vi "Main Test.vi"() -> ()   [LabVIEW 2020]
uses:
  Mete.ctl
  R.ctl
  P.ctl
  N.ctl
  D.ctl
  STOP.ctl
  Odo Velocity.ctl
  Gas.ctl
  Set-.ctl
  Set+.ctl
  Cru.ctl
  Dis.ctl
  CharRPM.ctl
  CharODO.ctl
  Brake.ctl
  Limit.ctl
  SET+LIMIT.ctl
  SET-LIMIT.ctl
panel:
  out "Image":T1(plugin-control)
  out "Boolean":T2
  in  "LIMIT-":T3
  in  "LIMT+":T4
  in  "LIMIT":T5
  in  "Slide 4":T6 scale=0.0..700.0
  out "Waveform Chart":T7
  out "Waveform Chart 2":T8
  in  "Dis":T9 caption="Boolean 8"
  in  "Cu":T10 caption="Boolean 7"
  in  "+Cu":T11 caption="Boolean 5"
  in  "-Cu":T12 caption="Boolean 6"
  in  "Slide 2":T13 scale=0.0..700.0
  out "Km/h":T14 scale=0.0..250.0
  in  "stop":T15
  out "Boolean 4":T16
  out "Boolean 3":T17
  out "Boolean 2":T18
  out "Gauge":T19 scale=0.0..650.0
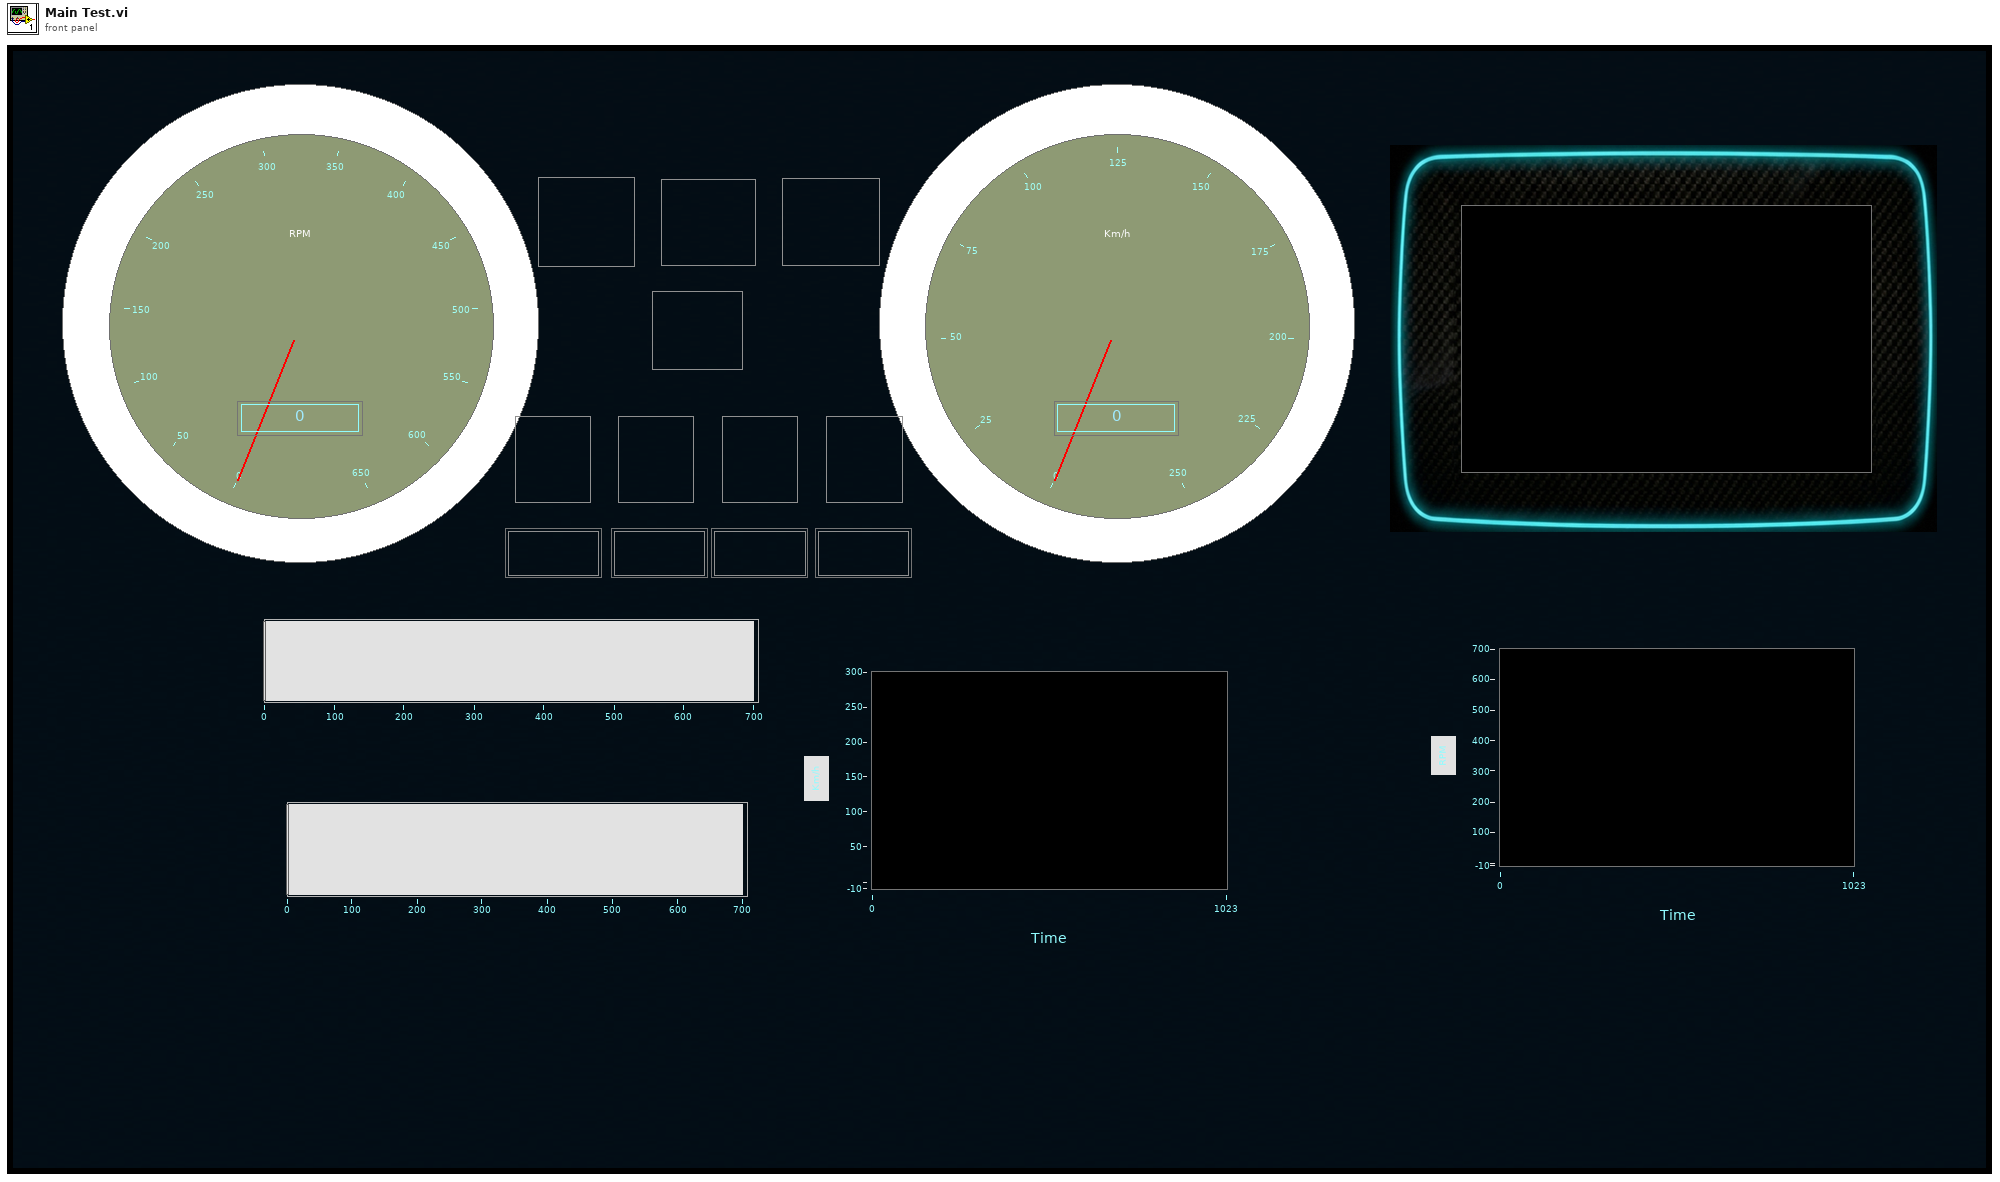
[diagram p1: front panel]
types:
  T1 = typedef "IMAQ Image.ctl" = refnum<image>
  T2 = typedef "R.ctl" = bool
  T3 = typedef "SET-LIMIT.ctl" = bool
  T4 = typedef "SET+LIMIT.ctl" = bool
  T5 = typedef "Limit.ctl" = bool
  T6 = typedef "Brake.ctl" = dbl
  T7 = typedef "CharODO.ctl" = dbl
  T8 = typedef "CharRPM.ctl" = dbl
  T9 = typedef "Dis.ctl" = bool
  T10 = typedef "Cru.ctl" = bool
  T11 = typedef "Set+.ctl" = bool
  T12 = typedef "Set-.ctl" = bool
  T13 = typedef "Gas.ctl" = dbl
  T14 = typedef "Odo Velocity.ctl" = u16
  T15 = typedef "STOP.ctl" = bool
  T16 = typedef "D.ctl" = bool
  T17 = typedef "N.ctl" = bool
  T18 = typedef "P.ctl" = bool
  T19 = typedef "Mete.ctl" = u16
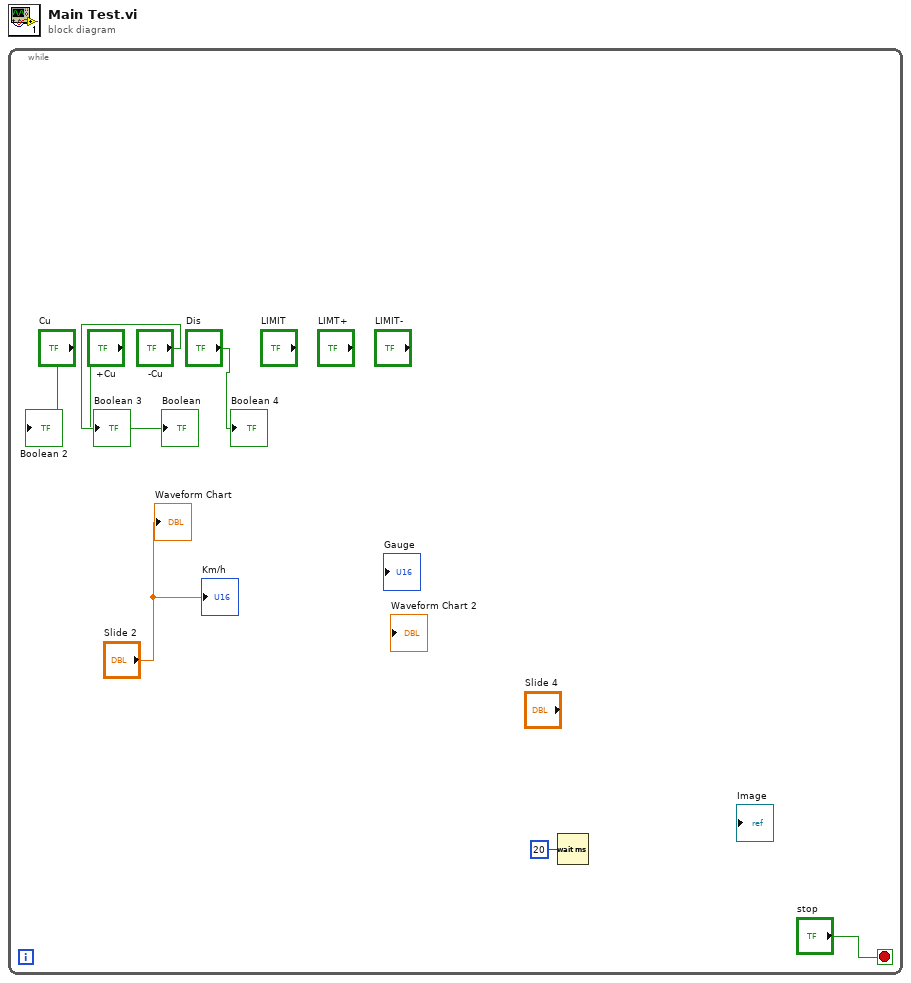
[diagram p0: block diagram]
diagram:
  n1 = while {
    stop <- "stop" stop-if-true
    n2 = Wait (ms)(milliseconds to wait=u32 20) -> ()  [unwired: 1 out]
    "Boolean 2" <- "Cu"
    "Boolean 3" <- "+Cu"
    "Boolean" <- "-Cu"
    "Boolean 4" <- "Dis"
    "Km/h" <- "Slide 2"
    "Waveform Chart" <- "Slide 2"
  }
